vi "PV_Core_Dlg_About.vi"   [LabVIEW 2020]
uses:
  <vilib>/event_ctls.llb/eventvkey.ctl
panel:
  # "PictureViewer"
types:
  T1 = enum32{"Invalid", "Standard", "Closed", "Hidden", "Minimized", "Maximized"}
  T2 = typedef "eventvkey.ctl" = enum16{"ASCII", "Enter", "Return", "Shift", "Ctrl", "Alt", "Cmd", "Opt", "Caps", "NumLock", "Clear", "Break", "Up", "Down", "Left", "Right", "Insert", "Delete", "Home", "End", "PageUp", "PageDown", "Escape", "Help", "Pause", "ScrollLock", "F1", "F2", "F3", "F4", "F5", "F6", "F7", "F8", "F9", "F10", "F11", "F12", "F13", "F14", "F15", "F16", "F17", "F18", "F19", "F20", "F21", "F22", "F23", "F24", "Play", "VolumeUp", "VolumeDown", "Mute", "Two Byte Char"}
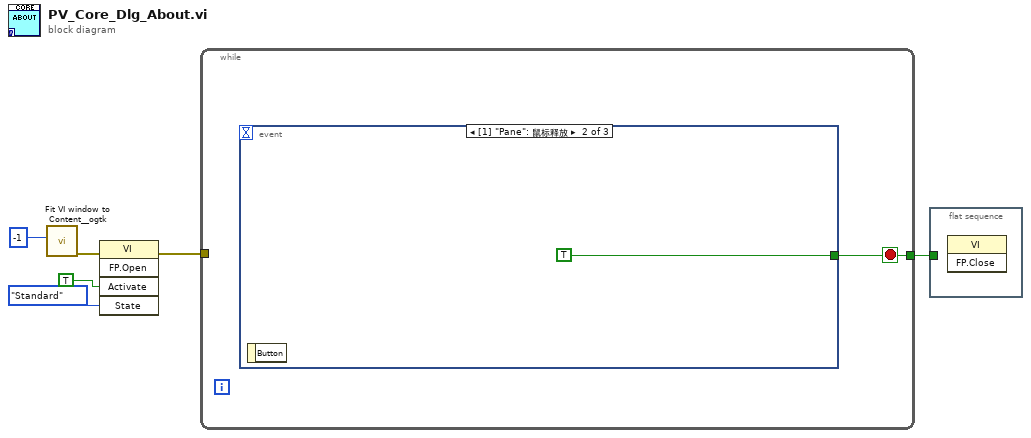
[diagram p0: block diagram]
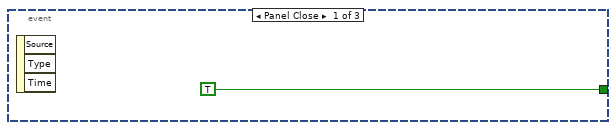
[diagram p2: hidden frame]
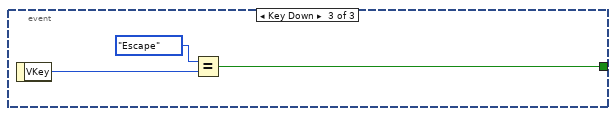
[diagram p3: hidden frame]
diagram:
  n1 = call <userlib>:"Fit VI window to Content__ogtk.vi"("border spacing (2 px)"=-1) -> ("error out"=w2:errorcluster)  [unwired: 5 in, 1 out]
  n2 = invoke class="VI" method="FP.Open"(error in=w2, "Activate"=TRUE ("Activate?"), "State"=T1."Standard") -> (error out=w1:errorcluster)  [unwired: 2 in, 4 out]
  n3 = while {
    tunnel: [w7] -> w6
    tunnel: w1 -> [_]
    stop <- w7 stop-if-true
    n4 = event shown="[1] \"Pane\": 鼠标释放" {
      selector: _ -> [_ _ _]
      dyn-events: _ -> [_ _ _]
      timeout: _ -> [_ _ _]
      tunnel: [TRUE TRUE w10] -> w7
      event Panel Close {
        n5 = event-data() -> ()  [unwired: 4 out]
      }
      event Mouse Up {
        n6 = event-data() -> ()  [unwired: 2 out]
      }
      event Key Down {
        n7 = event-data() -> ("VKey"=w11:T2)  [unwired: 1 out]
        n8 = Equal?(x=eventvkey."Escape" ("VKey"), y=w11) -> (x = y?=w10:bool)
      }
    }
  }
  n9 = flat-sequence {
    tunnel: w6 -> [_]
    frame #0 {
      n10 = invoke class="VI" method="FP.Close"() -> ()  [unwired: 3 in, 3 out]
    }
  }
